vi "Dresden R2R Sputter 03.02.2018 IY24.vi"() -> ()   [LabVIEW 2009] (continued)
        n5317 = call-poly <vilib>:"Draw Unflattened Pixmap.vi"("picture"=w7956, "top left point(0, 0)"=cluster{"x":i16, "y":i16} {"x"=484, "y"=640} ("top left point(0, 0) 2"), "data (RGB format)"=w7949) -> ("new picture"=w7941:picture)  [unwired: 6 in]
        n5318 = call-poly <vilib>:"Draw Unflattened Pixmap.vi"("picture"=w7941, "top left point(0, 0)"=cluster{"x":i16, "y":i16} {"x"=204, "y"=618} ("top left point(0, 0) 2"), "data (RGB format)"=w7948) -> ("new picture"=w7933:picture)  [unwired: 6 in]
        n5319 = call-poly <vilib>:"Draw Unflattened Pixmap.vi"("picture"=w7933, "top left point(0, 0)"=cluster{"x":i16, "y":i16} {"x"=279, "y"=625} ("top left point(0, 0) 2"), "data (RGB format)"=w7934) -> ("new picture"=w7925:picture)  [unwired: 6 in]
        n5320 = call-poly <vilib>:"Draw Unflattened Pixmap.vi"("picture"=w7925, "top left point(0, 0)"=cluster{"x":i16, "y":i16} {"x"=381, "y"=673} ("top left point(0, 0) 2"), "data (RGB format)"=w7926) -> ("new picture"=w7917:picture)  [unwired: 6 in]
        n5321 = call-poly <vilib>:"Draw Unflattened Pixmap.vi"("picture"=w7917, "top left point(0, 0)"=cluster{"x":i16, "y":i16} {"x"=370, "y"=635} ("top left point(0, 0) 2"), "data (RGB format)"=w7924) -> ("new picture"=w7909:picture)  [unwired: 6 in]
        n5322 = call-poly <vilib>:"Draw Unflattened Pixmap.vi"("picture"=w7909, "top left point(0, 0)"=cluster{"x":i16, "y":i16} {"x"=494, "y"=284} ("top left point(0, 0) 2"), "data (RGB format)"=w7910) -> ("new picture"=w7901:picture)  [unwired: 6 in]
        n5323 = call-poly <vilib>:"Draw Unflattened Pixmap.vi"("picture"=w7901, "top left point(0, 0)"=cluster{"x":i16, "y":i16} {"x"=512, "y"=205} ("top left point(0, 0) 2"), "data (RGB format)"=w7908) -> ("new picture"=w7856:picture)  [unwired: 6 in]
        n5324 = call-poly <vilib>:"Draw Unflattened Pixmap.vi"("picture"=w7856, "top left point(0, 0)"=cluster{"x":i16, "y":i16} {"x"=182, "y"=282}, "data (RGB format)"=w7866) -> ("new picture"=w7857:picture)  [unwired: 6 in]
      }
      frame #1 {
        n5325 = property on="new picture 6" class="Pict"() -> ("Mouse"=w8156:T37)  [unwired: 2 in, 2 out]
        n5326 = Unbundle(w8156) -> ("Mouse Position"=w8155:cluster{"X":i32, "Y":i32}, "Mouse Modifiers"=w8157:T38)
        "Mouse Position 7" <- w8155
        n5327 = Unbundle(w8157) -> ("Button Down"=w8135:bool)  [unwired: 3 out]
        n5328 = Unbundle(w8155) -> ("X"=w8018:i32, "Y"=w8019:i32)
        n5329 = In Range and Coerce(upper limit=595, x=w8019, lower limit=354) -> (In Range?=w8143:bool)  [unwired: 1 out]
        n5330 = In Range and Coerce(upper limit=619, x=w8018, lower limit=579) -> (In Range?=w8142:bool)  [unwired: 1 out]
        n5331 = In Range and Coerce(upper limit=596, x=w8019, lower limit=359) -> (In Range?=w8083:bool)  [unwired: 1 out]
        n5332 = In Range and Coerce(upper limit=146, x=w8018, lower limit=106) -> (In Range?=w8084:bool)  [unwired: 1 out]
        n5333 = In Range and Coerce(upper limit=670, x=w8019, lower limit=636) -> (In Range?=w8081:bool)  [unwired: 1 out]
        n5334 = In Range and Coerce(upper limit=315, x=w8018, lower limit=278) -> (In Range?=w8082:bool)  [unwired: 1 out]
        n5335 = In Range and Coerce(upper limit=254, x=w8019, lower limit=204) -> (In Range?=w8067:bool)  [unwired: 1 out]
        n5336 = In Range and Coerce(upper limit=536, x=w8018, lower limit=513) -> (In Range?=w8068:bool)  [unwired: 1 out]
        n5337 = In Range and Coerce(upper limit=674, x=w8019, lower limit=648) -> (In Range?=w8088:bool)  [unwired: 1 out]
        n5338 = In Range and Coerce(upper limit=530, x=w8018, lower limit=484) -> (In Range?=w8087:bool)  [unwired: 1 out]
        n5339 = In Range and Coerce(upper limit=391, x=w8019, lower limit=171) -> (In Range?=w8021:bool)  [unwired: 1 out]
        n5340 = In Range and Coerce(upper limit=652, x=w8019, lower limit=626) -> (In Range?=w8090:bool)  [unwired: 1 out]
        n5341 = In Range and Coerce(upper limit=705, x=w8019, lower limit=682) -> (In Range?=w8092:bool)  [unwired: 1 out]
        n5342 = In Range and Coerce(upper limit=381, x=w8018, lower limit=339) -> (In Range?=w8022:bool)  [unwired: 1 out]
        n5343 = In Range and Coerce(upper limit=229, x=w8018, lower limit=204) -> (In Range?=w8089:bool)  [unwired: 1 out]
        n5344 = In Range and Coerce(upper limit=406, x=w8018, lower limit=381) -> (In Range?=w8091:bool)  [unwired: 1 out]
        n5345 = In Range and Coerce(upper limit=367, x=w8019, lower limit=216) -> (In Range?=w8032:bool)  [unwired: 1 out]
        n5346 = In Range and Coerce(upper limit=367, x=w8019, lower limit=216) -> (In Range?=w8031:bool)  [unwired: 1 out]
        n5347 = In Range and Coerce(upper limit=310, x=w8019, lower limit=285) -> (In Range?=w8086:bool)  [unwired: 1 out]
        n5348 = In Range and Coerce(upper limit=305, x=w8018, lower limit=255) -> (In Range?=w8033:bool)  [unwired: 1 out]
        n5349 = In Range and Coerce(upper limit=463, x=w8018, lower limit=409) -> (In Range?=w8030:bool)  [unwired: 1 out]
        n5350 = In Range and Coerce(upper limit=228, x=w8018, lower limit=191) -> (In Range?=w8085:bool)  [unwired: 1 out]
        n5351 = In Range and Coerce(upper limit=243, x=w8019, lower limit=198) -> (In Range?=w8042:bool)  [unwired: 1 out]
        n5352 = In Range and Coerce(upper limit=595, x=w8018, lower limit=564) -> (In Range?=w8043:bool)  [unwired: 1 out]
        n5353 = In Range and Coerce(upper limit=312, x=w8019, lower limit=287) -> (In Range?=w8077:bool)  [unwired: 1 out]
        n5354 = In Range and Coerce(upper limit=531, x=w8018, lower limit=493) -> (In Range?=w8078:bool)  [unwired: 1 out]
        n5355 = In Range and Coerce(upper limit=660, x=w8019, lower limit=636) -> (In Range?=w8079:bool)  [unwired: 1 out]
        n5356 = In Range and Coerce(upper limit=407, x=w8018, lower limit=370) -> (In Range?=w8080:bool)  [unwired: 1 out]
        n5357 = And(x=w8084, y=w8083) -> (x .and. y?=w8152:bool)
        n5358 = And(x=w8142, y=w8143) -> (x .and. y?=w8148:bool)
        n5359 = And(x=w8082, y=w8081) -> (x .and. y?=w8153:bool)
        n5360 = And(x=w8022, y=w8021) -> (x .and. y?=w8015:bool)
        n5361 = And(x=w8080, y=w8079) -> (x .and. y?=w8154:bool)
        n5362 = And(x=w8033, y=w8032) -> (x .and. y?=w8017:bool)
        n5363 = And(x=w8030, y=w8031) -> (x .and. y?=w8016:bool)
        n5364 = And(x=w8078, y=w8077) -> (x .and. y?=w8133:bool)
        n5365 = And(x=w8089, y=w8090) -> (x .and. y?=w8129:bool)
        n5366 = And(x=w8068, y=w8067) -> (x .and. y?=w8132:bool)
        n5367 = And(x=w8085, y=w8086) -> (x .and. y?=w8131:bool)
        n5368 = And(x=w8087, y=w8088) -> (x .and. y?=w8130:bool)
        n5369 = And(x=w8091, y=w8092) -> (x .and. y?=w8128:bool)
        n5370 = And(x=w8043, y=w8042) -> (x .and. y?=w8038:bool)
        n5371 = And(x=w8135, y=w8148) -> (x .and. y?=w8146:bool)
        n5372 = And(x=w8135, y=w8152) -> (x .and. y?=w8149:bool)
        n5373 = And(x=w8135, y=w8153) -> (x .and. y?=w8150:bool)
        n5374 = And(x=w8135, y=w8133) -> (x .and. y?=w8137:bool)
        n5375 = And(x=w8135, y=w8132) -> (x .and. y?=w8136:bool)
        n5376 = And(x=w8135, y=w8131) -> (x .and. y?=w8134:bool)
        n5377 = And(x=w8135, y=w8154) -> (x .and. y?=w8151:bool)
        n5378 = case shown="True" w8146 {
          frame #0 {
          }
          frame #1 {
            "gv_top_timer_ch2_1" <- TRUE ("gv_top_timer_ch2_3")
          }
        }
        n5379 = case shown="True" w8149 {
          frame #0 {
          }
          frame #1 {
            "gv_top_timer_ch2_3" <- TRUE ("gv_top_timer_ch2_12")
          }
        }
        n5380 = case shown="True" w8151 {
          frame #0 {
          }
          frame #1 {
            "ch2_bg_bv_timer_top" <- TRUE ("ch2_cc_timer_top")
          }
        }
        n5381 = case shown="True" w8150 {
          frame #0 {
          }
          frame #1 {
            "ch2_cc_timer_top" <- TRUE ("ch2_cc_timer_top")
          }
        }
        n5382 = case shown="True" w8137 {
          frame #0 {
          }
          frame #1 {
            "ch2_ch_trns_gv_bp_timer_top" <- TRUE ("ch2_cc_timer_top")
          }
        }
        n5383 = case shown="True" w8136 {
          frame #0 {
          }
          frame #1 {
            "ch2_sov_Ar_timer_top" <- TRUE ("ch2_cc_timer_top")
          }
        }
        n5384 = case shown="True" w8134 {
          frame #0 {
          }
          frame #1 {
            "ch2_trns_gv_bp2_timer_top" <- TRUE ("ch2_cc_timer_top")
          }
        }
        n5385 = Build Array(TRUE, w8148, w8152, w8153, w8154, w8133, w8132, w8131, w8130, w8129, w8128, w8038, w8017, w8016, w8015) -> (w8145:bool[])
        n5386 = local read "ch2_trns_gv_bp2_timer_top"() -> (w8048:bool)
        n5387 = local read "ch2_ch_trns_gv_bp_timer_top"() -> (w8047:bool)
        n5388 = local read "ch2_bg_bv_timer_top"() -> (w8049:bool)
        n5389 = Boolean Array To Number(Boolean array=w8145) -> (number=w8144:u32)
        n5390 = local read "ch2_sov_Ar_timer_top"() -> (w8046:bool)
        n5391 = local read "gv_top_timer_ch2_3"() -> (w8051:bool)
        n5392 = local read "gv_top_timer_ch2_1"() -> (w8052:bool)
        n5393 = local read "ch2_cc_timer_top"() -> (w8050:bool)
        n5394 = Mantissa & Exponent(0:w8144) -> (2:w8076:dbl)  [unwired: 1 out]
        n5395 = case shown="14" w8076 {
          tunnel: [cluster{"x":i16, "y":i16} {"x"=0, "y"=0} ("origin") cluster{"x":i16, "y":i16} {"x"=633, "y"=472} ("origin") cluster{"x":i16, "y":i16} {"x"=73, "y"=465} ("origin") cluster{"x":i16, "y":i16} {"x"=281, "y"=678} ("origin") cluster{"x":i16, "y":i16} {"x"=413, "y"=647} ("origin") cluster{"x":i16, "y":i16} {"x"=511, "y"=270} ("origin") cluster{"x":i16, "y":i16} {"x"=507, "y"=187} ("origin") cluster{"x":i16, "y":i16} {"x"=186, "y"=268} ("origin") cluster{"x":i16, "y":i16} {"x"=490, "y"=686} ("origin") cluster{"x":i16, "y":i16} {"x"=209, "y"=659} ("origin") cluster{"x":i16, "y":i16} {"x"=380, "y"=716} ("origin") cluster{"x":i16, "y":i16} {"x"=560, "y"=180} ("origin") cluster{"x":i16, "y":i16} {"x"=257, "y"=167} ("origin") cluster{"x":i16, "y":i16} {"x"=411, "y"=167} ("origin") cluster{"x":i16, "y":i16} {"x"=329, "y"=149} ("origin")] -> w8073
          tunnel: ["" ("text") "GV" ("text") "GV" ("text") "CH-CC" ("text") "BG-BV" ("text") "GV-BP" ("text") "SOV-Ar" ("text") "GV-BP" ("text") "CH-ATM" ("text") "CH-PG" ("text") "CH-BG" ("text") "MFC" ("text") "CST-FIX" ("text") "CST-FIX" ("text") "PET-COOL" ("text")] -> w8074
          tunnel: ["" ("DESCRIPTION") "Gate Valve" ("DESCRIPTION") "Gate Valve" ("DESCRIPTION") "Chamber-Cold Cathode" ("DESCRIPTION") "Baratron Gauge-Block Valve" ("DESCRIPTION") "Gate Valve- By Pass" ("DESCRIPTION") "Shut Off Valve-Ar Gas" ("DESCRIPTION") "Gate Valve- By Pass" ("DESCRIPTION") "Chamber-Atmospheric Switch" ("DESCRIPTION") "Chamber-Pirani Gauge" ("DESCRIPTION") "Chamber-Baratron Gauge" ("DESCRIPTION") "Mass Flow Control" ("DESCRIPTION") "Casette Fix" ("DESCRIPTION") "Casette Fix" ("DESCRIPTION") "Petfolio Cool " ("DESCRIPTION")] -> w8075
          frame #0 {
          }
          frame #1 {
          }
          frame #2 {
          }
          frame #3 {
          }
          frame #4 {
          }
          frame #5 {
          }
          frame #6 {
          }
          frame #7 {
          }
          frame #8 {
          }
          frame #9 {
          }
          frame #10 {
          }
          frame #11 {
          }
          frame #12 {
          }
          frame #13 {
          }
          frame #14 {
          }
        }
        n5396 = feedback #151() -> (w8057:bool)  [unwired: 1 in]
        n5397 = feedback #152() -> (w8065:bool)  [unwired: 1 in]
        n5398 = feedback #153() -> (w8064:bool)  [unwired: 1 in]
        n5399 = feedback #154() -> (w8061:bool)  [unwired: 1 in]
        n5400 = feedback #155() -> (w8060:bool)  [unwired: 1 in]
        n5401 = feedback #156() -> (w8056:bool)  [unwired: 1 in]
        n5402 = feedback #157() -> (w8053:bool)  [unwired: 1 in]
        n5403 = case shown="True" w8048 {
          tunnel: [TRUE FALSE] -> w8058
          tunnel: w8057 -> [_ w8186]
          frame #0 {
          }
          frame #1 {
            n5404 = call "Elapsed Time75"("Reset"=w8186) -> ("Elapsed Time (s)"=w8183:dbl)  [unwired: 11 in, 7 out]
            n5405 = Greater?(x=w8183, y=3.0) -> (0:w8184:bool)
            n5406 = In Range and Coerce(upper limit=3.0, x=w8183, lower limit=0.0) -> (In Range?=w8180:bool)  [unwired: 1 out]
            n5407 = Not(x=w8184) -> (.not. x?=w8179:bool)
            n5408 = local write "ch2_trns_gv_bp2_timer_top"(w8179) -> ()
            n5409 = property on="Ch2_trns_gv_bp2_timer_top_gui" class="TabCtl (strict)"("Visible"=w8180) -> ()  [unwired: 2 in, 2 out]
          }
        }
        n5410 = case shown="True" w8052 {
          tunnel: [TRUE FALSE] -> w8066
          tunnel: w8065 -> [_ w8226]
          frame #0 {
          }
          frame #1 {
            n5411 = call "Elapsed Time71"("Reset"=w8226) -> ("Elapsed Time (s)"=w8223:dbl)  [unwired: 11 in, 7 out]
            n5412 = Greater?(x=w8223, y=3.0) -> (0:w8224:bool)
            n5413 = In Range and Coerce(upper limit=3.0, x=w8223, lower limit=0.0) -> (In Range?=w8219:bool)  [unwired: 1 out]
            n5414 = Not(x=w8224) -> (.not. x?=w8220:bool)
            n5415 = local write "gv_top_timer_ch2_1"(w8220) -> ()
            n5416 = property on="Gv_timer_top_ch2_1_gui" class="TabCtl (strict)"("Visible"=w8219) -> ()  [unwired: 2 in, 2 out]
          }
        }
        n5417 = case shown="True" w8051 {
          tunnel: [TRUE FALSE] -> w8063
          tunnel: w8064 -> [_ w8216]
          frame #0 {
          }
          frame #1 {
            n5418 = call "Elapsed Time72"("Reset"=w8216) -> ("Elapsed Time (s)"=w8213:dbl)  [unwired: 11 in, 7 out]
            n5419 = Greater?(x=w8213, y=3.0) -> (0:w8214:bool)
            n5420 = In Range and Coerce(upper limit=3.0, x=w8213, lower limit=0.0) -> (In Range?=w8209:bool)  [unwired: 1 out]
            n5421 = Not(x=w8214) -> (.not. x?=w8210:bool)
            n5422 = local write "gv_top_timer_ch2_3"(w8210) -> ()
            n5423 = property on="Gv_timer_top_ch2_3_gui" class="TabCtl (strict)"("Visible"=w8209) -> ()  [unwired: 2 in, 2 out]
          }
        }
        n5424 = case shown="True" w8050 {
          tunnel: [TRUE FALSE] -> w8062
          tunnel: w8061 -> [_ w8206]
          frame #0 {
          }
          frame #1 {
            n5425 = call "Elapsed Time73"("Reset"=w8206) -> ("Elapsed Time (s)"=w8203:dbl)  [unwired: 11 in, 7 out]
            n5426 = Greater?(x=w8203, y=3.0) -> (0:w8204:bool)
            n5427 = In Range and Coerce(upper limit=3.0, x=w8203, lower limit=0.0) -> (In Range?=w8200:bool)  [unwired: 1 out]
            n5428 = Not(x=w8204) -> (.not. x?=w8199:bool)
            n5429 = local write "ch2_cc_timer_top"(w8199) -> ()
            n5430 = property on="Ch2_cc_timer_top_gui" class="TabCtl (strict)"("Visible"=w8200) -> ()  [unwired: 2 in, 2 out]
          }
        }
        n5431 = case shown="True" w8049 {
          tunnel: [TRUE FALSE] -> w8059
          tunnel: w8060 -> [_ w8196]
          frame #0 {
          }
          frame #1 {
            n5432 = call "Elapsed Time74"("Reset"=w8196) -> ("Elapsed Time (s)"=w8193:dbl)  [unwired: 11 in, 7 out]
            n5433 = Greater?(x=w8193, y=3.0) -> (0:w8194:bool)
            n5434 = In Range and Coerce(upper limit=3.0, x=w8193, lower limit=0.0) -> (In Range?=w8190:bool)  [unwired: 1 out]
            n5435 = Not(x=w8194) -> (.not. x?=w8189:bool)
            n5436 = local write "ch2_bg_bv_timer_top"(w8189) -> ()
            n5437 = property on="Ch2_bg_bv_timer_top_gui" class="TabCtl (strict)"("Visible"=w8190) -> ()  [unwired: 2 in, 2 out]
          }
        }
        n5438 = case shown="True" w8047 {
          tunnel: [TRUE FALSE] -> w8055
          tunnel: w8056 -> [_ w8176]
          frame #0 {
          }
          frame #1 {
            n5439 = call "Elapsed Time76"("Reset"=w8176) -> ("Elapsed Time (s)"=w8173:dbl)  [unwired: 11 in, 7 out]
            n5440 = Greater?(x=w8173, y=3.0) -> (0:w8174:bool)
            n5441 = In Range and Coerce(upper limit=3.0, x=w8173, lower limit=0.0) -> (In Range?=w8169:bool)  [unwired: 1 out]
            n5442 = Not(x=w8174) -> (.not. x?=w8170:bool)
            n5443 = local write "ch2_ch_trns_gv_bp_timer_top"(w8170) -> ()
            n5444 = property on="Ch2_trns_gv_bp_timer_top_gui" class="TabCtl (strict)"("Visible"=w8169) -> ()  [unwired: 2 in, 2 out]
          }
        }
        n5445 = case shown="True" w8046 {
          tunnel: [TRUE FALSE] -> w8054
          tunnel: w8053 -> [_ w8166]
          frame #0 {
          }
          frame #1 {
            n5446 = call "Elapsed Time77"("Reset"=w8166) -> ("Elapsed Time (s)"=w8163:dbl)  [unwired: 11 in, 7 out]
            n5447 = Greater?(x=w8163, y=3.0) -> (0:w8164:bool)
            n5448 = In Range and Coerce(upper limit=3.0, x=w8163, lower limit=0.0) -> (In Range?=w8160:bool)  [unwired: 1 out]
            n5449 = Not(x=w8164) -> (.not. x?=w8159:bool)
            n5450 = local write "ch2_sov_Ar_timer_top"(w8159) -> ()
            n5451 = property on="Ch2_sov_Ar_timer_top_gui" class="TabCtl (strict)"("Visible"=w8160) -> ()  [unwired: 2 in, 2 out]
          }
        }
        n5452 = local write "DESCRIPTION"(w8075) -> ()
        n5453 = call <vilib>:"Draw Text at Point.vi"("[user-specified font]"=T35 {"Font Name:"="BOLD", "Size"=18, "Strikeout?"=FALSE, "Italic?"=FALSE, "Underline?"=FALSE, "Outline?"=FALSE, "Shadow?"=FALSE, "Bold?"=TRUE} ("[user-specified font] 7"), "desired font(Application)"=T36."User-specified Font", "text"=w8074, "origin"=w8073, "picture"=w8072) -> ("new picture"=w8071:picture)  [unwired: 5 in, 1 out]
      }
    }
    "new picture 6" <- w7814
    n5454 = Wait Until Next ms Multiple(millisecond multiple=u32 100) -> ()  [unwired: 1 out]
  }
  n5455 = VISA Close(VISA resource name=w15, error in (no error)=w14) -> ()  [unwired: 1 out]
  n5456 = while {
    stop <- FALSE stop-if-true
    n5457 = Wait Until Next ms Multiple(millisecond multiple=u32 300) -> ()  [unwired: 1 out]
    n5458 = case shown="True" "Start_full_foil" {
      frame #0 {
      }
      frame #1 {
        n5459 = case shown="\"Specified Length of Foil\"" "Roll_Selection" {
          frame #0 {
            n5460 = local read "Chamber_selection_roll"() -> (w8551:T14)
            n5461 = case shown="\"Chamber 4\"" w8551 {
              frame #0 {
                n5462 = stacked-sequence {
                  frame #0 {
                    n5463 = local read "Max Diameter 2"() -> (w8556:dbl)
                    n5464 = local read "Min Diameter 2"() -> (w8555:dbl)
                    n5465 = local read "Web_Thickness2"() -> (w8552:dbl)
                    n5466 = local read "Web Speed 2"() -> (w8553:dbl)
                    n5467 = local write "Max Diameter"(w8556) -> ()
                    n5468 = local write "Min Diameter"(w8555) -> ()
                    n5469 = local write "Web Speed"(w8553) -> ()
                    n5470 = local write "Web Thickness"(w8552) -> ()
                    n5471 = Wait (ms)(milliseconds to wait=u32 1000) -> ()  [unwired: 1 out]
                  }
                  frame #1 {
                    n5472 = local write "Calculate_auto"(TRUE ("Calculate_auto")) -> ()
                    n5473 = Wait (ms)(milliseconds to wait=u32 300) -> ()  [unwired: 1 out]
                  }
                  frame #2 {
                    w8559 = u16 0 items=["1", "2", "3", "4"] ("Target Chamber Sensor")
                    n5474 = local write "Target Chamber Sensor"(w8559) -> ()
                  }
                  frame #3 {
                    n5475 = local read "Roll_side_select 2"() -> (w8560:enum32{"Left to Right", "Right to Left"})
                    n5476 = case shown="\"Right to Left\"" w8560 {
                      frame #0 {
                        n5477 = local read "Tension_Value2"() -> (w8563:dbl)
                        n5478 = local write "TC1_set_value"(w8563) -> ()
                        n5479 = Wait (ms)(milliseconds to wait=u32 300) -> ()  [unwired: 1 out]
                        n5480 = local write "Roll_side_select"(enum32{"Left to Right", "Right to Left"}."Left to Right" ("Roll_side_select")) -> ()
                      }
                      frame #1 {
                        n5481 = local read "Tension_Value2"() -> (w8566:dbl)
                        n5482 = local write "TC2_set_value"(w8566) -> ()
                        n5483 = local write "Roll_side_select"(enum32{"Left to Right", "Right to Left"}."Right to Left" ("Roll_side_select")) -> ()
                        n5484 = Wait (ms)(milliseconds to wait=u32 300) -> ()  [unwired: 1 out]
                      }
                    }
                  }
                  frame #4 {
                    n5485 = local read "Roll_side_select 2"() -> (w8567:enum32{"Left to Right", "Right to Left"})
                    n5486 = case shown="\"Left to Right\", Default" w8567 {
                      frame #0 {
                        n5487 = local write "TC1_set"(TRUE ("TC1_set")) -> ()
                      }
                      frame #1 {
                        n5488 = local write "TC2_set"(TRUE ("TC2_set")) -> ()
                      }
                    }
                  }
                  frame #5 {
                    n5489 = local write "Parameters_auto_set"(TRUE ("Parameters_auto_set")) -> ()
                    n5490 = Wait (ms)(milliseconds to wait=u32 1000) -> ()  [unwired: 1 out]
                  }
                  frame #6 {
                    n5491 = while {
                      i -> [w8577]
                      stop <- w8572 stop-if-true
                      n5492 = Greater?(x=w8577, y=100) -> (0:w8573:bool)
                      n5493 = Wait Until Next ms Multiple(millisecond multiple=u32 300) -> ()  [unwired: 1 out]
                      n5494 = local read "Parameters_auto_set"() -> (w8578:bool)
                      n5495 = case shown="True" w8578 {
                        tunnel: [TRUE FALSE] -> w8574
                        frame #0 {
                        }
                        frame #1 {
                        }
                      }
                      n5496 = Or(x=w8574, y=w8573) -> (x .or. y?=w8572:bool)
                    }
                  }
                  frame #7 {
                    n5497 = local write "Start_roll"(TRUE ("Start_roll")) -> ()
                  }
                  frame #8 {
                    n5498 = while {
                      stop <- w8585 stop-if-true
                      n5499 = local read "Actual Length"() -> (w8589:dbl)
                      n5500 = local read "Region"() -> (w8588:dbl)
                      n5501 = local read "Start_full_foil"() -> (w8583:bool)
                      n5502 = local read "Semi"() -> (w8586:bool)
                      n5503 = Greater Or Equal?(x=w8589, y=w8588) -> (x >= y?=w8587:bool)
                      n5504 = Not(x=w8583) -> (.not. x?=w8582:bool)
                      n5505 = Compound Arithmetic op=OR(w8582, w8587, w8586) -> (w8585:bool)
                      n5506 = Wait Until Next ms Multiple(millisecond multiple=u32 300) -> ()  [unwired: 1 out]
                    }
                  }
                  frame #9 {
                    n5507 = local write "Start_full_foil"(FALSE ("Start_full_foil")) -> ()
                  }
                }
              }
              frame #1 {
                n5508 = stacked-sequence {
                  frame #0 {
                    n5509 = local read "Max Diameter 2"() -> (w8595:dbl)
                    n5510 = local read "Min Diameter 2"() -> (w8594:dbl)
                    n5511 = local read "Web_Thickness2"() -> (w8591:dbl)
                    n5512 = local read "Web Speed 2"() -> (w8592:dbl)
                    n5513 = local write "Max Diameter"(w8595) -> ()
                    n5514 = local write "Min Diameter"(w8594) -> ()
                    n5515 = local write "Web Speed"(w8592) -> ()
                    n5516 = local write "Web Thickness"(w8591) -> ()
                    n5517 = Wait (ms)(milliseconds to wait=u32 1000) -> ()  [unwired: 1 out]
                  }
                  frame #1 {
                    n5518 = local write "Calculate_auto"(TRUE ("Calculate_auto")) -> ()
                    n5519 = Wait (ms)(milliseconds to wait=u32 1000) -> ()  [unwired: 1 out]
                  }
                  frame #2 {
                    w8598 = u16 1 items=["1", "2", "3", "4"] ("Target Chamber Sensor")
                    n5520 = local write "Target Chamber Sensor"(w8598) -> ()
                  }
                  frame #3 {
                    n5521 = local read "Roll_side_select 2"() -> (w8599:enum32{"Left to Right", "Right to Left"})
                    n5522 = case shown="\"Right to Left\"" w8599 {
                      frame #0 {
                        n5523 = local read "Tension_Value2"() -> (w8602:dbl)
                        n5524 = local write "Roll_side_select"(enum32{"Left to Right", "Right to Left"}."Left to Right" ("Roll_side_select")) -> ()
                        n5525 = local write "TC1_set_value"(w8602) -> ()
                        n5526 = Wait (ms)(milliseconds to wait=u32 300) -> ()  [unwired: 1 out]
                      }
                      frame #1 {
                        n5527 = local read "Tension_Value2"() -> (w8605:dbl)
                        n5528 = local write "TC2_set_value"(w8605) -> ()
                        n5529 = local write "Roll_side_select"(enum32{"Left to Right", "Right to Left"}."Right to Left" ("Roll_side_select")) -> ()
                        n5530 = Wait (ms)(milliseconds to wait=u32 300) -> ()  [unwired: 1 out]
                      }
                    }
                  }
                  frame #4 {
                    n5531 = local read "Roll_side_select 2"() -> (w8606:enum32{"Left to Right", "Right to Left"})
                    n5532 = case shown="\"Left to Right\", Default" w8606 {
                      frame #0 {
                        n5533 = local write "TC1_set"(TRUE ("TC1_set")) -> ()
                      }
                      frame #1 {
                        n5534 = local write "TC2_set"(TRUE ("TC2_set")) -> ()
                      }
                    }
                  }
                  frame #5 {
                    n5535 = local write "Parameters_auto_set"(TRUE ("Parameters_auto_set")) -> ()
                    n5536 = Wait (ms)(milliseconds to wait=u32 1000) -> ()  [unwired: 1 out]
                  }
                  frame #6 {
                    n5537 = while {
                      i -> [w8616]
                      stop <- w8611 stop-if-true
                      n5538 = Greater?(x=w8616, y=100) -> (0:w8612:bool)
                      n5539 = Wait Until Next ms Multiple(millisecond multiple=u32 300) -> ()  [unwired: 1 out]
                      n5540 = local read "Parameters_auto_set"() -> (w8617:bool)
                      n5541 = case shown="False" w8617 {
                        tunnel: [TRUE FALSE] -> w8613
                        frame #0 {
                        }
                        frame #1 {
                        }
                      }
                      n5542 = Or(x=w8613, y=w8612) -> (x .or. y?=w8611:bool)
                    }
                  }
                  frame #7 {
                    n5543 = local write "Start_roll"(TRUE ("Start_roll")) -> ()
                  }
                  frame #8 {
                    n5544 = while {
                      stop <- w8622 stop-if-true
                      n5545 = local read "Actual Length"() -> (w8626:dbl)
                      n5546 = local read "Region"() -> (w8625:dbl)
                      n5547 = local read "Semi"() -> (w8623:bool)
                      n5548 = Greater Or Equal?(x=w8626, y=w8625) -> (x >= y?=w8624:bool)
                      n5549 = Or(x=w8624, y=w8623) -> (x .or. y?=w8622:bool)
                      n5550 = Wait Until Next ms Multiple(millisecond multiple=u32 300) -> ()  [unwired: 1 out]
                    }
                  }
                  frame #9 {
                    n5551 = local write "Start_full_foil"(FALSE ("Start_full_foil")) -> ()
                  }
                }
              }
              frame #2 {
                n5552 = stacked-sequence {
                  frame #0 {
                    n5553 = local read "Max Diameter 2"() -> (w8632:dbl)
                    n5554 = local read "Min Diameter 2"() -> (w8631:dbl)
                    n5555 = local read "Web_Thickness2"() -> (w8628:dbl)
                    n5556 = local read "Web Speed 2"() -> (w8629:dbl)
                    n5557 = local write "Max Diameter"(w8632) -> ()
                    n5558 = local write "Min Diameter"(w8631) -> ()
                    n5559 = local write "Web Thickness"(w8628) -> ()
                    n5560 = local write "Web Speed"(w8629) -> ()
                    n5561 = Wait (ms)(milliseconds to wait=u32 1000) -> ()  [unwired: 1 out]
                  }
                  frame #1 {
                    n5562 = local write "Calculate_auto"(TRUE ("Calculate_auto")) -> ()
                    n5563 = Wait (ms)(milliseconds to wait=u32 1000) -> ()  [unwired: 1 out]
                  }
                  frame #2 {
                    w8636 = u16 2 items=["1", "2", "3", "4"] ("Target Chamber Sensor")
                    n5564 = local write "Target Chamber Sensor"(w8636) -> ()
                    n5565 = Wait (ms)(milliseconds to wait=u32 1000) -> ()  [unwired: 1 out]
                  }
                  frame #3 {
                    n5566 = local read "Roll_side_select 2"() -> (w8637:enum32{"Left to Right", "Right to Left"})
                    n5567 = case shown="\"Right to Left\"" w8637 {
                      frame #0 {
                        n5568 = local read "Tension_Value2"() -> (w8640:dbl)
                        n5569 = local write "Roll_side_select"(enum32{"Left to Right", "Right to Left"}."Left to Right" ("Roll_side_select")) -> ()
                        n5570 = local write "TC1_set_value"(w8640) -> ()
                        n5571 = Wait (ms)(milliseconds to wait=u32 300) -> ()  [unwired: 1 out]
                      }
                      frame #1 {
                        n5572 = local read "Tension_Value2"() -> (w8643:dbl)
                        n5573 = local write "TC2_set_value"(w8643) -> ()
                        n5574 = local write "Roll_side_select"(enum32{"Left to Right", "Right to Left"}."Right to Left" ("Roll_side_select")) -> ()
                        n5575 = Wait (ms)(milliseconds to wait=u32 300) -> ()  [unwired: 1 out]
                      }
                    }
                  }
                  frame #4 {
                    n5576 = local read "Roll_side_select 2"() -> (w8644:enum32{"Left to Right", "Right to Left"})
                    n5577 = case shown="\"Left to Right\", Default" w8644 {
                      frame #0 {
                        n5578 = local write "TC1_set"(TRUE ("TC1_set")) -> ()
                      }
                      frame #1 {
                        n5579 = local write "TC2_set"(TRUE ("TC2_set")) -> ()
                      }
                    }
                  }
                  frame #5 {
                    n5580 = local write "Parameters_auto_set"(TRUE ("Parameters_auto_set")) -> ()
                    n5581 = Wait (ms)(milliseconds to wait=u32 1000) -> ()  [unwired: 1 out]
                  }
                  frame #6 {
                    n5582 = while {
                      i -> [w8654]
                      stop <- w8649 stop-if-true
                      n5583 = Greater?(x=w8654, y=100) -> (0:w8650:bool)
                      n5584 = Wait Until Next ms Multiple(millisecond multiple=u32 300) -> ()  [unwired: 1 out]
                      n5585 = local read "Parameters_auto_set"() -> (w8655:bool)
                      n5586 = case shown="False" w8655 {
                        tunnel: [TRUE FALSE] -> w8651
                        frame #0 {
                        }
                        frame #1 {
                        }
                      }
                      n5587 = Or(x=w8651, y=w8650) -> (x .or. y?=w8649:bool)
                    }
                  }
                  frame #7 {
                    n5588 = local write "Start_roll"(TRUE ("Start_roll")) -> ()
                  }
                  frame #8 {
                    n5589 = while {
                      stop <- w8660 stop-if-true
                      n5590 = local read "Actual Length"() -> (w8664:dbl)
                      n5591 = local read "Region"() -> (w8663:dbl)
                      n5592 = local read "Semi"() -> (w8661:bool)
                      n5593 = Greater Or Equal?(x=w8664, y=w8663) -> (x >= y?=w8662:bool)
                      n5594 = Or(x=w8662, y=w8661) -> (x .or. y?=w8660:bool)
                      n5595 = Wait Until Next ms Multiple(millisecond multiple=u32 300) -> ()  [unwired: 1 out]
                    }
                  }
                  frame #9 {
                    n5596 = local write "Start_full_foil"(FALSE ("Start_full_foil")) -> ()
                  }
                }
              }
              frame #3 {
                n5597 = stacked-sequence {
                  frame #0 {
                    n5598 = local read "Max Diameter 2"() -> (w8670:dbl)
                    n5599 = local read "Min Diameter 2"() -> (w8669:dbl)
                    n5600 = local read "Web_Thickness2"() -> (w8666:dbl)
                    n5601 = local read "Web Speed 2"() -> (w8667:dbl)
                    n5602 = local write "Max Diameter"(w8670) -> ()
                    n5603 = local write "Min Diameter"(w8669) -> ()
                    n5604 = local write "Web Thickness"(w8666) -> ()
                    n5605 = local write "Web Speed"(w8667) -> ()
                    n5606 = Wait (ms)(milliseconds to wait=u32 1000) -> ()  [unwired: 1 out]
                  }
                  frame #1 {
                    n5607 = local write "Calculate_auto"(TRUE ("Calculate_auto")) -> ()
                    n5608 = Wait (ms)(milliseconds to wait=u32 1000) -> ()  [unwired: 1 out]
                  }
                  frame #2 {
                    w8674 = u16 3 items=["1", "2", "3", "4"] ("Target Chamber Sensor")
                    n5609 = local write "Target Chamber Sensor"(w8674) -> ()
                    n5610 = Wait (ms)(milliseconds to wait=u32 1000) -> ()  [unwired: 1 out]
                  }
                  frame #3 {
                    n5611 = local read "Roll_side_select 2"() -> (w8675:enum32{"Left to Right", "Right to Left"})
                    n5612 = case shown="\"Right to Left\"" w8675 {
                      frame #0 {
                        n5613 = local read "Tension_Value2"() -> (w8678:dbl)
                        n5614 = local write "Roll_side_select"(enum32{"Left to Right", "Right to Left"}."Left to Right" ("Roll_side_select")) -> ()
                        n5615 = local write "TC1_set_value"(w8678) -> ()
                        n5616 = Wait (ms)(milliseconds to wait=u32 300) -> ()  [unwired: 1 out]
                      }
                      frame #1 {
                        n5617 = local read "Tension_Value2"() -> (w8681:dbl)
                        n5618 = local write "TC2_set_value"(w8681) -> ()
                        n5619 = local write "Roll_side_select"(enum32{"Left to Right", "Right to Left"}."Right to Left" ("Roll_side_select")) -> ()
                        n5620 = Wait (ms)(milliseconds to wait=u32 300) -> ()  [unwired: 1 out]
                      }
                    }
                  }
                  frame #4 {
                    n5621 = local read "Roll_side_select 2"() -> (w8682:enum32{"Left to Right", "Right to Left"})
                    n5622 = case shown="\"Right to Left\"" w8682 {
                      frame #0 {
                        n5623 = local write "TC1_set"(TRUE ("TC1_set")) -> ()
                      }
                      frame #1 {
                        n5624 = local write "TC2_set"(TRUE ("TC2_set")) -> ()
                      }
                    }
                  }
                  frame #5 {
                    n5625 = local write "Parameters_auto_set"(TRUE ("Parameters_auto_set")) -> ()
                    n5626 = Wait (ms)(milliseconds to wait=u32 1000) -> ()  [unwired: 1 out]
                  }
                  frame #6 {
                    n5627 = while {
                      i -> [w8692]
                      stop <- w8687 stop-if-true
                      n5628 = Greater?(x=w8692, y=100) -> (0:w8688:bool)
                      n5629 = Wait Until Next ms Multiple(millisecond multiple=u32 300) -> ()  [unwired: 1 out]
                      n5630 = local read "Parameters_auto_set"() -> (w8693:bool)
                      n5631 = case shown="False" w8693 {
                        tunnel: [TRUE FALSE] -> w8689
                        frame #0 {
                        }
                        frame #1 {
                        }
                      }
                      n5632 = Or(x=w8689, y=w8688) -> (x .or. y?=w8687:bool)
                    }
                  }
                  frame #7 {
                    n5633 = local write "Start_roll"(TRUE ("Start_roll")) -> ()
                  }
                  frame #8 {
                    n5634 = while {
                      stop <- w8698 stop-if-true
                      n5635 = local read "Actual Length"() -> (w8702:dbl)
                      n5636 = local read "Region"() -> (w8701:dbl)
                      n5637 = local read "Semi"() -> (w8699:bool)
                      n5638 = Greater Or Equal?(x=w8702, y=w8701) -> (x >= y?=w8700:bool)
                      n5639 = Or(x=w8700, y=w8699) -> (x .or. y?=w8698:bool)
                      n5640 = Wait Until Next ms Multiple(millisecond multiple=u32 300) -> ()  [unwired: 1 out]
                    }
                  }
                  frame #9 {
                    n5641 = local write "Start_full_foil"(FALSE ("Start_full_foil")) -> ()
                  }
                }
              }
            }
          }
          frame #1 {
            n5642 = local read "Chamber_selection_roll"() -> (w8704:T14)
            n5643 = case shown="\"Chamber 3\"" w8704 {
              frame #0 {
                n5644 = local read "Roll_side_select 2"() -> (w8705:enum32{"Left to Right", "Right to Left"})
                n5645 = case shown="\"Right to Left\"" w8705 {
                  frame #0 {
                    n5646 = stacked-sequence {
                      frame #0 {
                        n5647 = local read "Target_length_left side"() -> (w8709:dbl)
                        n5648 = local read "Web_Thickness2"() -> (w8706:dbl)
                        n5649 = local read "Max Diameter 2"() -> (w8712:dbl)
                        n5650 = local read "Min Diameter 2"() -> (w8711:dbl)
                        n5651 = local read "Web Speed 2"() -> (w8707:dbl)
                        n5652 = local write "Initial Min Diameter"(w8711) -> ()
                        n5653 = local write "Web Speed"(w8707) -> ()
                        n5654 = local write "Max Diameter"(w8712) -> ()
                        n5655 = local write "Roll_side_select"(enum32{"Left to Right", "Right to Left"}."Left to Right" ("Roll_side_select")) -> ()
                        n5656 = local write "Web Thickness"(w8706) -> ()
                        n5657 = local write "Region"(w8709) -> ()
                        n5658 = Wait (ms)(milliseconds to wait=u32 1000) -> ()  [unwired: 1 out]
                      }
                      frame #1 {
                        n5659 = local write "Calculate 2"(TRUE ("Calculate_auto")) -> ()
                      }
                      frame #2 {
                        n5660 = local read "Tension_Value2"() -> (w8715:dbl)
                        n5661 = Wait (ms)(milliseconds to wait=u32 300) -> ()  [unwired: 1 out]
                        n5662 = local write "TC1_set_value"(w8715) -> ()
                      }
                      frame #3 {
                        w8716 = u16 0 items=["1", "2", "3", "4"] ("Target Chamber Sensor")
                        n5663 = local write "Target Chamber Sensor"(w8716) -> ()
                      }
                      frame #4 {
                        n5664 = local write "TC1_set"(TRUE ("TC1_set")) -> ()
                      }
                      frame #5 {
                        n5665 = local write "Parameters_auto_set"(TRUE ("Parameters_auto_set")) -> ()
                      }
                      frame #6 {
                        n5666 = while {
                          i -> [w8724]
                          stop <- w8719 stop-if-true
                          n5667 = Greater?(x=w8724, y=100) -> (0:w8720:bool)
                          n5668 = Wait Until Next ms Multiple(millisecond multiple=u32 300) -> ()  [unwired: 1 out]
                          n5669 = local read "Parameters_auto_set"() -> (w8725:bool)
                          n5670 = case shown="False" w8725 {
                            tunnel: [TRUE FALSE] -> w8721
                            frame #0 {
                            }
                            frame #1 {
                            }
                          }
                          n5671 = Or(x=w8721, y=w8720) -> (x .or. y?=w8719:bool)
                        }
                      }
                      frame #7 {
                        n5672 = local write "Start_roll"(TRUE ("Start_roll")) -> ()
                      }
                      frame #8 {
                        n5673 = while {
                          stop <- w8730 stop-if-true
                          n5674 = local read "Actual Length"() -> (w8734:dbl)
                          n5675 = local read "Region"() -> (w8733:dbl)
                          n5676 = local read "Semi"() -> (w8731:bool)
                          n5677 = Greater Or Equal?(x=w8734, y=w8733) -> (x >= y?=w8732:bool)
                          n5678 = Or(x=w8732, y=w8731) -> (x .or. y?=w8730:bool)
                          n5679 = Wait Until Next ms Multiple(millisecond multiple=u32 300) -> ()  [unwired: 1 out]
                        }
                      }
                      frame #9 {
                        n5680 = local write "Start_full_foil"(FALSE ("Start_full_foil")) -> ()
                      }
                    }
                  }
                  frame #1 {
                    n5681 = stacked-sequence {
                      frame #0 {
                        n5682 = local read "Target_length_right side"() -> (w8740:dbl)
                        n5683 = local read "Web_Thickness2"() -> (w8736:dbl)
                        n5684 = local read "Max Diameter 2"() -> (w8741:dbl)
                        n5685 = local read "Web Speed 2"() -> (w8737:dbl)
                        n5686 = local write "Web Speed"(w8737) -> ()
                        n5687 = local write "Web Thickness"(w8736) -> ()
                        n5688 = local write "Max Diameter"(w8741) -> ()
                        n5689 = local write "Roll_side_select"(enum32{"Left to Right", "Right to Left"}."Right to Left" ("Roll_side_select")) -> ()
                        n5690 = local write "Region"(w8740) -> ()
                        n5691 = Wait (ms)(milliseconds to wait=u32 1000) -> ()  [unwired: 1 out]
                      }
                      frame #1 {
                        n5692 = local write "Calculate 3"(TRUE ("Calculate_auto")) -> ()
                      }
                      frame #2 {
                        n5693 = local read "Change_Max Diameter"() -> (w8744:dbl)
                        n5694 = Wait (ms)(milliseconds to wait=u32 300) -> ()  [unwired: 1 out]
                        n5695 = local write "Initial Min Diameter"(w8744) -> ()
                      }
                      frame #3 {
                        n5696 = local write "Calculate 2"(TRUE ("Calculate_auto")) -> ()
                      }
                      frame #4 {
                        w8746 = u16 0 items=["1", "2", "3", "4"] ("Target Chamber Sensor")
                        n5697 = local write "Target Chamber Sensor"(w8746) -> ()
                      }
                      frame #5 {
                        n5698 = local read "Tension_Value2"() -> (w8748:dbl)
                        n5699 = Wait (ms)(milliseconds to wait=u32 300) -> ()  [unwired: 1 out]
                        n5700 = local write "TC2_set_value"(w8748) -> ()
                      }
                      frame #6 {
                        n5701 = local write "TC2_set"(TRUE ("TC1_set")) -> ()
                      }
                      frame #7 {
                        n5702 = local write "Parameters_auto_set"(TRUE ("Parameters_auto_set")) -> ()
                      }
                      frame #8 {